vi "UHR-Fleezers Control (host) - 12.7e.vi"() -> ()   [LabVIEW 2012] (continued)
        n866 = flat-sequence {
          tunnel: w1282 -> [w1285]
          frame #0 {
            # "set paramaters (rate, volume) for flush, clear volume"
            n867 = Number To Decimal String(number="Flush rate (uL/m) P3") -> (decimal integer string=w1307:string)  [unwired: 1 in]
            n868 = local write "Inject Pump 3"(TRUE ("Inject Pump 3")) -> ()
            n869 = Concatenate Strings("irate  " ("string"), w1307, " u/m" ("string"), "\r") -> (w1309:string)
            n870 = VISA Write(VISA resource name=w1285, write buffer=w1309) -> (VISA resource name out=w1305:refnum<visa-resource-name>)  [unwired: 1 in, 2 out]
            n871 = Reciprocal(x="Flush rate (uL/m) P3") -> (1/x=w1289:dbl)
            n872 = Number To Decimal String(number="Volume (uL) P3") -> (decimal integer string=w1296:string)  [unwired: 1 in]
            n873 = Multiply(x="Volume (uL) P3", y=w1289) -> (x*y=w1288:dbl)
            n874 = Concatenate Strings("tvolume  " ("string"), w1296, " u" ("string"), "\r") -> (w1294:string)
            n875 = Multiply(x=w1288, y=60.0) -> (x*y=→"HP3 Flush Time (s)":dbl)
            n876 = VISA Write(VISA resource name=w1305, write buffer=w1294) -> (VISA resource name out=w1293:refnum<visa-resource-name>)  [unwired: 1 in, 2 out]
            n877 = Concatenate Strings("cvolume" ("string"), "\r") -> (w1292:string)
            n878 = VISA Write(VISA resource name=w1293, write buffer=w1292) -> (VISA resource name out=w1303:refnum<visa-resource-name>)  [unwired: 1 in, 2 out]
            n879 = Concatenate Strings("irun" ("string"), "\r") -> (w1301:string)
            n880 = VISA Write(VISA resource name=w1303, write buffer=w1301) -> ()  [unwired: 1 in, 3 out]
          }
          frame #1 {
            "Flushing P3" <- TRUE ("Flushing P3")
          }
        }
      }
      event "Flush Pump 1": Value Change {
        n881 = event-data() -> ()  [unwired: 7 out]
        n882 = flat-sequence {
          tunnel: [w1323] -> w1313
          tunnel: w1312 -> [w1316]
          tunnel: w1313 -> [_]
          frame #0 {
            # "set paramaters (rate, volume) for flush, clear volume"
            n883 = local write "Inject Pump 1"(TRUE ("Inject Pump 1")) -> ()
            n884 = Number To Decimal String(number="Flush rate (uL/m) P1") -> (decimal integer string=w1339:string)  [unwired: 1 in]
            n885 = Concatenate Strings("irate  " ("string"), w1339, " u/m" ("string"), "\r") -> (w1341:string)
            n886 = VISA Write(VISA resource name=w1316, write buffer=w1341) -> (VISA resource name out=w1337:refnum<visa-resource-name>)  [unwired: 1 in, 2 out]
            n887 = Reciprocal(x="Flush rate (uL/m) P1") -> (1/x=w1320:dbl)
            n888 = Number To Decimal String(number="Volume (uL) P1") -> (decimal integer string=w1328:string)  [unwired: 1 in]
            n889 = Multiply(x="Volume (uL) P1", y=w1320) -> (x*y=w1319:dbl)
            n890 = Concatenate Strings("tvolume  " ("string"), w1328, " u" ("string"), "\r") -> (w1326:string)
            n891 = Multiply(x=w1319, y=60.0) -> (x*y=→"HP1 Flush Time (s)":dbl)
            n892 = VISA Write(VISA resource name=w1337, write buffer=w1326) -> (VISA resource name out=w1325:refnum<visa-resource-name>)  [unwired: 1 in, 2 out]
            n893 = Concatenate Strings("cvolume" ("string"), "\r") -> (w1324:string)
            n894 = VISA Write(VISA resource name=w1325, write buffer=w1324) -> (VISA resource name out=w1335:refnum<visa-resource-name>)  [unwired: 1 in, 2 out]
            n895 = Concatenate Strings("irun" ("string"), "\r") -> (w1333:string)
            n896 = VISA Write(VISA resource name=w1335, write buffer=w1333) -> (VISA resource name out=w1323:refnum<visa-resource-name>)  [unwired: 1 in, 2 out]
          }
          frame #1 {
            "Flushing P1" <- TRUE ("Flushing P3")
          }
        }
      }
      event "Clear Volume": Value Change {
        n897 = event-data() -> ()  [unwired: 7 out]
        n898 = Concatenate Strings("cvolume" ("string"), "\r") -> (w1345:string)
        n899 = VISA Write(VISA resource name=w1344, write buffer=w1345) -> ()  [unwired: 1 in, 3 out]
      }
      event "Clear Volume P3": Value Change {
        n900 = event-data() -> ()  [unwired: 7 out]
        n901 = Concatenate Strings("cvolume" ("string"), "\r") -> (w1351:string)
        n902 = VISA Write(VISA resource name=w1350, write buffer=w1351) -> ()  [unwired: 1 in, 3 out]
        n903 = local write "Clear Volume P3"(FALSE ("Clear Volume P3")) -> ()
      }
      event "Clear Volume P1": Value Change {
        n904 = event-data() -> ()  [unwired: 7 out]
        n905 = Concatenate Strings("cvolume" ("string"), "\r") -> (w1356:string)
        n906 = local write "Clear Volume P1"(FALSE ("Clear Volume P1")) -> ()
        n907 = VISA Write(VISA resource name=w1355, write buffer=w1356) -> ()  [unwired: 1 in, 3 out]
      }
      event "Display On P3": Value Change {
        n908 = event-data() -> ()  [unwired: 7 out]
        n909 = Select(t="dim 100", s="Display On P3", f="dim 0") -> (s? t:f=w1362:string)
        n910 = Concatenate Strings(w1362, "\r") -> (w1364:string)
        n911 = VISA Write(VISA resource name=w1359, write buffer=w1364) -> ()  [unwired: 1 in, 3 out]
      }
      event "Display On P1": Value Change {
        n912 = event-data() -> ()  [unwired: 7 out]
        n913 = Select(t="dim 100", s="Display On P1", f="dim 0") -> (s? t:f=w1369:string)
        n914 = Concatenate Strings(w1369, "\r") -> (w1371:string)
        n915 = VISA Write(VISA resource name=w1366, write buffer=w1371) -> ()  [unwired: 1 in, 3 out]
      }
      event "Retract Pump 3": Value Change {
        n916 = event-data() -> ()  [unwired: 7 out]
        n917 = local write "Retract Pump 3"(FALSE ("Retract Pump 3")) -> ()
        n918 = case shown="True" "Retract Pump 3" {
          tunnel: w1373 -> [_ w1376]
          frame False {
          }
          frame True {
            n919 = Number To Decimal String(number="Retract Rate (uL/m)") -> (decimal integer string=w1394:string)  [unwired: 1 in]
            n920 = Concatenate Strings("wrate  " ("string"), w1394, " u/m" ("string"), "\r") -> (w1396:string)
            n921 = VISA Write(VISA resource name=w1376, write buffer=w1396) -> (VISA resource name out=w1387:refnum<visa-resource-name>)  [unwired: 1 in, 2 out]
            n922 = Number To Decimal String(number="Retract Vol 3 (uL)") -> (decimal integer string=w1389:string)  [unwired: 1 in]
            n923 = Concatenate Strings("tvolume  " ("string"), w1389, " u" ("string"), "\r") -> (w1386:string)
            n924 = VISA Write(VISA resource name=w1387, write buffer=w1386) -> (VISA resource name out=w1382:refnum<visa-resource-name>)  [unwired: 1 in, 2 out]
            n925 = Concatenate Strings("cvolume" ("string"), "\r") -> (w1383:string)
            n926 = VISA Write(VISA resource name=w1382, write buffer=w1383) -> (VISA resource name out=w1377:refnum<visa-resource-name>)  [unwired: 1 in, 2 out]
            n927 = Concatenate Strings("wrun" ("string"), "\r") -> (w1378:string)
            n928 = VISA Write(VISA resource name=w1377, write buffer=w1378) -> ()  [unwired: 1 in, 3 out]
          }
        }
      }
      event "Retract Pump 1": Value Change {
        n929 = event-data() -> ()  [unwired: 7 out]
        n930 = local write "Retract Pump 1"(FALSE ("Retract Pump 1")) -> ()
        n931 = case shown="True" "Retract Pump 1" {
          tunnel: w1398 -> [_ w1403]
          frame False {
          }
          frame True {
            n932 = local read "Retract Rate (uL/m)"() -> (w1401:dbl)
            n933 = Number To Decimal String(number=w1401) -> (decimal integer string=w1419:string)  [unwired: 1 in]
            n934 = Concatenate Strings("wrate  " ("string"), w1419, " u/m" ("string"), "\r") -> (w1421:string)
            n935 = VISA Write(VISA resource name=w1403, write buffer=w1421) -> (VISA resource name out=w1413:refnum<visa-resource-name>)  [unwired: 1 in, 2 out]
            n936 = Number To Decimal String(number="Retract Vol 1 (uL)") -> (decimal integer string=w1415:string)  [unwired: 1 in]
            n937 = Concatenate Strings("tvolume  " ("string"), w1415, " u" ("string"), "\r") -> (w1412:string)
            n938 = VISA Write(VISA resource name=w1413, write buffer=w1412) -> (VISA resource name out=w1409:refnum<visa-resource-name>)  [unwired: 1 in, 2 out]
            n939 = Concatenate Strings("cvolume" ("string"), "\r") -> (w1410:string)
            n940 = VISA Write(VISA resource name=w1409, write buffer=w1410) -> (VISA resource name out=w1404:refnum<visa-resource-name>)  [unwired: 1 in, 2 out]
            n941 = Concatenate Strings("wrun" ("string"), "\r") -> (w1405:string)
            n942 = VISA Write(VISA resource name=w1404, write buffer=w1405) -> ()  [unwired: 1 in, 3 out]
          }
        }
      }
      event "Flip Green Filter": Value Change {
        n943 = event-data() -> ()  [unwired: 7 out]
        n944 = Not(x="Flip Green Filter") -> (.not. x?=w1424:bool)
        n945 = local write "Flip Green Filter"(w1424) -> ()
        n946 = flat-sequence {
          tunnel: [w1433] -> w1429
          tunnel: [w1432] -> w1428
          tunnel: w1423 -> [w1431]
          tunnel: [w1436] -> w1427
          tunnel: w1429 -> [w1436]
          tunnel: [w1435] -> w1426
          tunnel: w1428 -> [w1435]
          tunnel: w1427 -> [w1440]
          tunnel: w1426 -> [w1439]
          tunnel: [w1438] -> w1430
          frame #0 {
            n947 = xnode "Read/Write Control"("FPGA VI Reference In"=w1431, "Green Filter Flipper"=TRUE) -> ("FPGA VI Reference Out"=w1433:T20, "error out"=w1432:errorcluster)  [unwired: 1 in]
          }
          frame #1 {
            n948 = Wait (ms)(milliseconds to wait=u32 100) -> ()  [unwired: 1 out]
          }
          frame #2 {
            n949 = xnode "Read/Write Control"("FPGA VI Reference In"=w1440, "error in"=w1439, "Green Filter Flipper"=FALSE) -> ("error out"=w1438:errorcluster)  [unwired: 1 out]
          }
        }
      }
      event "Pump 1 contents", "Pump 3 contents": Value Change {
        n950 = event-data() -> ()  [unwired: 7 out]
        n951 = local read "Pump 1 contents"() -> (→"Pump 1 cont disp":string)
        n952 = local read "Pump 3 contents"() -> (→"Pump 3 cont disp":string)
      }
      event "Reset Trap Pos. FB": Value Change {
        n953 = event-data() -> ()  [unwired: 7 out]
        n954 = xnode "Read/Write Control"("FPGA VI Reference In"=w1444, "Trap Pos. FB Reset"="Reset Trap Pos. FB") -> ()  [unwired: 1 in, 2 out]
      }
      event "Rem fb disp offset": Value Change {
        n955 = event-data() -> ()  [unwired: 7 out]
        n956 = local write "Rem fb disp offset"(FALSE ("Rem fb disp offset")) -> ()
        n957 = local read "Mean T1 Position (nm)"() -> (w1447:dbl)
        n958 = local read "FB Trap Pos Offset"() -> (w1448:dbl)
        n959 = Subtract(x=w1448, y=w1447) -> (x-y=w1446:dbl)
        n960 = local write "FB Trap Pos Offset"(w1446) -> ()
      }
      event "Threshold (nm)": Value Change {
        n961 = event-data() -> ()  [unwired: 7 out]
        n962 = flat-sequence {
          tunnel: [w1453] -> w1451
          tunnel: w1450 -> [w1452]
          tunnel: w1451 -> [w1464]
          frame #0 {
            n963 = xnode "Read/Write Control"("FPGA VI Reference In"=w1452) -> ("FPGA VI Reference Out"=w1456:T20, "error out"=w1455:errorcluster, "FPGA TTrig Thresh"=w1457:i64)  [unwired: 1 in]
            n964 = local read "Threshold stored (nm)"() -> (w1463:dbl)
            n965 = local read "Threshold (nm)"() -> (w1453:dbl)
            n966 = local read "AOM X Cal (nm/MHz)"() -> (w1461:dbl)
            n967 = Subtract(x=w1453, y=w1463) -> (x-y=w1462:dbl)
            n968 = Divide(x=w1462, y=w1461) -> (x/y=w1459:dbl)
            n969 = call "IR AOM freq to word.vi"("Frequency In (MHz)"=w1459) -> ("Frequency Word Out (double)"=w1460:dbl)
            n970 = To Quad Integer(1:w1460) -> (0:w1458:i64)
            n971 = Add(x=w1457, y=w1458) -> (x+y=w1454:i64)
            n972 = xnode "Read/Write Control"("FPGA VI Reference In"=w1456, "error in"=w1455, "FPGA TTrig Thresh"=w1454) -> ()  [unwired: 2 out]
          }
          frame #1 {
            "Threshold stored (nm)" <- w1464
          }
        }
      }
      event "FB Trig Integrate": Value Change {
        n973 = event-data() -> ()  [unwired: 7 out]
        n974 = local read "FB Trig Integrate"() -> (w1467:u32)
        n975 = xnode "Read/Write Control"("FPGA VI Reference In"=w1465, "FB Trig Integrate"=w1467) -> ("error out"=w1466:errorcluster)  [unwired: 1 in, 1 out]
      }
      event "11": Value Change {
        n976 = event-data() -> ()  [unwired: 7 out]
        n977 = local read "11"() -> (w1468:bool)
        n978 = case shown="True" w1468 {
          frame False {
          }
          frame True {
            n979 = local read "Messages"() -> (w1470:string)
            n980 = call "Update messages.vi"("Message to add"="You kicked it up to 11!", "Old message string"=w1470) -> ("New message string"=w1471:string)
            n981 = call <vilib>:"Beep.vi"() -> ()  [unwired: 12 in]
            n982 = local write "Messages"(w1471) -> ()
          }
        }
      }
      event "Trap Pos. FB ON": Value Change {
        n983 = event-data() -> ()  [unwired: 7 out]
        n984 = xnode "Read/Write Control"("FPGA VI Reference In"=w1472, "Force feedback"="Trap Pos. FB ON") -> ()  [unwired: 1 in, 2 out]
      }
      event "Remove Action Offset": Value Change {
        n985 = event-data() -> ()  [unwired: 7 out]
        n986 = local write "Remove Action Offset"(FALSE ("Remove Action Offset")) -> ()
        n987 = local read "Trap Pos. FB Mult Factor"() -> (w1479:i64)
        n988 = local read "Trap Pos FB Action"() -> (w1477:i64)
        n989 = local read "Trap Pos. FB Offset Factor"() -> (w1475:i64)
        n990 = Multiply(x=w1479, y=w1477) -> (x*y=w1478:i64)
        n991 = Add(x=w1478, y=w1475) -> (x+y=w1476:i64)
        n992 = local write "Trap Pos. FB Offset Factor"(w1476) -> ()
        n993 = xnode "Read/Write Control"("FPGA VI Reference In"=w1474, "Trap Pos. FB Offset Factor"=w1476) -> ()  [unwired: 1 in, 2 out]
      }
      event "Remove Unwinding Offset": Value Change {
        n994 = event-data() -> ()  [unwired: 7 out]
        n995 = local write "Remove Unwinding Offset"(FALSE ("Remove Action Offset")) -> ()
        n996 = local read "Trap Pos. FB Mult Factor"() -> (w1493:i64)
        n997 = local read "Trap Pos FB Action"() -> (w1491:i64)
        n998 = local read "Trap Pos. FB Offset Factor"() -> (w1490:i64)
        n999 = Multiply(x=w1493, y=w1491) -> (x*y=w1492:i64)
        n1000 = local read "Trap Pos. FB Mult Factor"() -> (w1489:i64)
        n1001 = Add(x=w1492, y=w1490) -> (x+y=w1483:i64)
        n1002 = Multiply(x=32768, y="factor") -> (x*y=w1486:dbl)
        n1003 = Multiply(x=w1486, y=w1489) -> (x*y=w1488:dbl)
        n1004 = Subtract(x=w1483, y=w1488) -> (x-y=w1487:dbl)
        n1005 = To Quad Integer(1:w1487) -> (0:w1482:i64)
        n1006 = xnode "Read/Write Control"("FPGA VI Reference In"=w1481, "Trap Pos. FB Offset Factor"=w1482) -> ()  [unwired: 1 in, 2 out]
        n1007 = local write "Trap Pos. FB Offset Factor"(w1482) -> ()
      }
      event "Trap Pos. FB Range", "Trap Pos. FB Gains", "Trap Pos. FB Mult Factor", "Trap Pos. FB Offset Factor", "Trap Pos FB Negate Action", "Trap Pos FB Monitor\nT1 or T2", "Differential FB?", "Negate Diff?": Value Change {
        n1008 = event-data() -> ()  [unwired: 7 out]
        n1009 = Unbundle By Name("Trap Pos. FB Gains") -> ("proportional gain (Kc)"=w1498:fxp<+/-,16,8>, "integral gain (Kc*Ts/Ti)"=w1497:fxp<+/-,16,8>, "derivative gain (Kc*Td/Ts)"=w1496:fxp<+/-,16,8>)
        n1010 = local read "Negate Diff?"() -> (w1503:bool)
        n1011 = Unbundle By Name("Trap Pos. FB Range") -> ("output high"=w1501:fxp<+/-,16,1>, "output low"=w1500:fxp<+/-,16,1>)
        n1012 = xnode "Read/Write Control"("FPGA VI Reference In"=w1495, "FB2 output high"=w1501, "FB2 output low"=w1500, "P2"=w1498, "I2"=w1497, "D2"=w1496, "Trap Pos. FB Mult Factor"="Trap Pos. FB Mult Factor", "Trap Pos. FB Offset Factor"="Trap Pos. FB Offset Factor", "Trap Pos FB Negate Action"="Trap Pos FB Negate Action", "Trap Pos FB Monitor T1 or T2"="Trap Pos FB Monitor\nT1 or T2", "AI1 X Scale"="Trap Pos. AI1 X Pre-scale", "Negate Diff?"=w1503, "Diff FB Measurement?"="Differential FB?") -> ()  [unwired: 1 in, 2 out]
      }
      event "Trap Pos FB SP", "Trap Pos FB SP 2", "Use SP 2": Value Change {
        n1013 = event-data() -> ()  [unwired: 7 out]
        n1014 = Select(t="Trap Pos FB SP 2", s="Use SP 2", f="Trap Pos FB SP") -> (s? t:f=w1511:fxp<+/-,16,1>)
        n1015 = xnode "Read/Write Control"("FPGA VI Reference In"=w1510, "Trap Pos. FB SP"=w1511) -> ()  [unwired: 1 in, 2 out]
      }
      event "Offset SP2 from SP1": Value Change {
        n1016 = event-data() -> ()  [unwired: 7 out]
        n1017 = local read "Trap Pos FB SP"() -> (w1517:fxp<+/-,16,1>)
        n1018 = Add(x=w1517, y="SP2 Offset") -> (x+y=w1515:fxp<+/-,16,1>)
        n1019 = property on="Trap Pos FB SP 2" class="DigNum (strict)"("Val(Sgnl)"=w1515) -> ()  [unwired: 2 in, 2 out]
        n1020 = local write "Offset SP2 from SP1"(FALSE ("Offset SP2 from SP1")) -> ()
      }
      event "Set Reading to\nSetpoint": Value Change {
        # "This is the actual PID input signal"
        n1021 = event-data() -> ()  [unwired: 7 out]
        n1022 = local write "Set Reading to\nSetpoint"(FALSE ("Set SP to Reading")) -> ()
        n1023 = xnode "Read/Write Control"("FPGA VI Reference In"=w1519) -> ("FPGA VI Reference Out"=w1522:T20, "error out"=w1521:errorcluster, "Trap Pos FB Int-Norm Signal"=w1520:fxp<+/-,16,1>)  [unwired: 1 in]
        n1024 = local read "Differential FB?"() -> (w1523:bool)
        n1025 = case shown="False" w1523 {
          tunnel: [w1528 w1535] -> w1525
          tunnel: w1520 -> [w1526 w1535]
          frame False {
            n1026 = local read "Trap Pos FB Monitor\nT1 or T2"() -> (w1531:bool)
            n1027 = local read "Trap X AI1 (DMA)"() -> (w1534:T13)
            n1028 = Unbundle By Name(w1534) -> ("Set 1"=w1533:fxp<+/-,16,1>, "Set 2"=w1532:fxp<+/-,16,1>)
            n1029 = Select(t=w1533, s=w1531, f=w1532) -> (s? t:f=w1530:fxp<+/-,16,1>)
            n1030 = Not(x="Set SP Using...") -> (.not. x?=w1527:bool)
            n1031 = Select(t=w1526, s=w1527, f=w1530) -> (s? t:f=w1528:fxp<+/-,16,1>)
          }
          frame True {
          }
        }
        n1032 = xnode "Read/Write Control"("FPGA VI Reference In"=w1522, "error in"=w1521, "Trap Pos. FB SP"=w1525) -> ()  [unwired: 2 out]
        n1033 = local write "Trap Pos FB SP"(w1525) -> ()
      }
      event "Trap Pos. FB Out Scale 2^n": Value Change {
        n1034 = event-data() -> ()  [unwired: 7 out]
        n1035 = Scale By Power Of 2(n="Trap Pos. FB Out Scale 2^n", x=ext 1.0) -> (x*2^n=w1536:ext)
        n1036 = property on="Trap Pos. FB Mult Factor" class="DigNum (strict)"("Val(Sgnl)"=w1536) -> ()  [unwired: 2 in, 2 out]
      }
      event "Trap Pos FB Int Count": Value Change {
        n1037 = event-data() -> ()  [unwired: 7 out]
        n1038 = xnode "Read/Write Control"("FPGA VI Reference In"=w1539, "Trap Pos FB Int Count"="Trap Pos FB Int Count") -> ()  [unwired: 1 in, 2 out]
      }
      event "Trap pos": Value Change {
        n1039 = event-data() -> ()  [unwired: 7 out]
        n1040 = case shown="True" "Trap pos" {
          frame False {
            n1041 = property on="Trap Delta Graph" class="WFGraph (strict)"("Visible"=TRUE) -> ()  [unwired: 2 in, 2 out]
            n1042 = property on="Saved trap pos" class="WFGraph (strict)"("Visible"=FALSE) -> ()  [unwired: 2 in, 2 out]
          }
          frame True {
            n1043 = property on="Saved trap pos" class="WFGraph (strict)"("Visible"=TRUE) -> ()  [unwired: 2 in, 2 out]
            n1044 = property on="Trap Delta Graph" class="WFGraph (strict)"("Visible"=FALSE) -> ()  [unwired: 2 in, 2 out]
          }
        }
      }
    }
    "error out 2" <- w406
    n1045 = node-c288() -> ()  [unwired: 2 out]
  }
  n1046 = timed-loop "Rough control of MCL mirror stage (debugging)" {
    tunnel: [w1548] -> w76
    timing: w22 -> [_]
    timing-out: [_] -> w21
    tunnel: w5 -> [w1546]
    stop <- w1548 stop-if-true
    n1047 = node-c288() -> ()  [unwired: 2 out]
    n1048 = case shown="2" "MCL Mode" {
      tunnel: w1546 -> [_ w1551 w1598]
      frame 0, Default {
      }
      frame 1 {
        n1049 = node-c288() -> (w1553:T23)  [unwired: 4 out]
        n1050 = timed-loop "Oscillate MCL mirror" {
          timing: w1553 -> [_]
          timing-out: [_] -> w1552
          tunnel: w1551 -> [w1554]
          i -> [w1592]
          stop <- w1555 stop-if-true
          n1051 = node-c288() -> (w1591:i64)  [unwired: 1 out]
          n1052 = Multiply(x="AO1", y=32767.0) -> (x*y=w1587:dbl)
          n1053 = Multiply(x="AO2", y=32767.0) -> (x*y=w1582:dbl)
          n1054 = Divide(x=w1587, y=10.0) -> (x/y=w1588:dbl)
          n1055 = Divide(x=w1582, y=10.0) -> (x/y=w1583:dbl)
          n1056 = To Word Integer(number=w1588) -> (16bit integer=w1580:i16)
          n1057 = To Word Integer(number=w1583) -> (16bit integer=w1579:i16)
          n1058 = Divide(x=w1591, y=i64 1000) -> (x/y=w1562:dbl)
          n1059 = Multiply(x=w1562, y=w1592) -> (x*y=w1573:dbl)
          n1060 = Multiply(x="Osc. freq. (Hz) 2", y=6.283185307179586) -> (x*y=w1574:dbl)
          n1061 = Multiply(x=w1574, y=w1573) -> (x*y=w1572:dbl)
          n1062 = Sine(x=w1572) -> (sin(x)=w1571:dbl)
          n1063 = Multiply(x=w1571, y="Osc. amp. (V)") -> (x*y=w1569:dbl)
          n1064 = Add(x=w1569, y="Osc. center (V)") -> (x+y=w1567:dbl)
          n1065 = Divide(x=w1567, y=10.0) -> (x/y=w1565:dbl)
          n1066 = Multiply(x=w1565, y=32767.0) -> (x*y=w1560:dbl)
          n1067 = Select(t=w1560, s="Scan axis", f=w1580) -> (s? t:f=w1578:dbl)
          n1068 = Select(t=w1579, s="Scan axis", f=w1560) -> (s? t:f=w1577:dbl)
          n1069 = local read "MCL Mode"() -> (w1559:u16)
          n1070 = Not Equal?(x=w1559, y=u16 1) -> (x != y?=w1556:bool)
          n1071 = local read "Stop All"() -> (w1557:bool)
          n1072 = xnode "Read/Write Control"("FPGA VI Reference In"=w1554, "AO1"=w1578, "AO2"=w1577) -> ()  [unwired: 1 in, 2 out]
          n1073 = Compound Arithmetic op=OR(w1557, w1556) -> (w1555:bool)
          n1074 = node-c288() -> ()  [unwired: 2 out]
        }
        n1075 = node-c288(w1552) -> ()  [unwired: 1 out]
      }
      frame 2 {
        n1076 = case shown="True" "Start Scan" {
          tunnel: w1598 -> [_ w1600]
          frame False {
          }
          frame True {
            n1077 = Subtract(x="End (V)", y="Begin (V)") -> (x-y=w1607:dbl)
            n1078 = Decrement(x="N Points") -> (x-1=w1606:dbl)
            n1079 = Divide(x=w1607, y=w1606) -> (x/y=w1604:dbl)
            n1080 = for {
              N: "N Points" -> [_]
              tunnel: "Begin (V)" -> [w1623]
              tunnel: [w1615] -> w1610 mode=indexing
              tunnel: w1604 -> [w1614]
              tunnel: [w1612] -> w1603 mode=indexing
              tunnel: w1600 -> [w1611]
              i -> [w1622]
              n1081 = Multiply(x=w1614, y=w1622) -> (x*y=w1621:dbl)
              n1082 = Add(x=w1623, y=w1621) -> (x+y=w1618:dbl)
              n1083 = local read "Scan axis"() -> (w1613:bool)
              n1084 = local read "AO1"() -> (w1620:dbl)
              n1085 = local read "AO2"() -> (w1619:dbl)
              n1086 = Select(t=w1618, s=w1613, f=w1620) -> (s? t:f=w1617:dbl)
              n1087 = Select(t=w1619, s=w1613, f=w1618) -> (s? t:f=w1616:dbl)
              n1088 = flat-sequence {
                tunnel: w1617 -> [w1627]
                tunnel: w1616 -> [w1626]
                tunnel: w1611 -> [w1624]
                tunnel: [w1637] -> w1615
                tunnel: [w1636] -> w1612
                frame #0 {
                  w1630 = 10.0 ("y")
                  w1625 = 32767.0 ("y")
                  n1089 = Multiply(x=w1627, y=w1625) -> (x*y=w1633:dbl)
                  n1090 = Multiply(x=w1626, y=w1625) -> (x*y=w1631:dbl)
                  n1091 = Divide(x=w1633, y=w1630) -> (x/y=w1634:dbl)
                  n1092 = Divide(x=w1631, y=w1630) -> (x/y=w1632:dbl)
                  n1093 = To Word Integer(number=w1634) -> (16bit integer=w1628:i16)
                  n1094 = To Word Integer(number=w1632) -> (16bit integer=w1629:i16)
                  n1095 = xnode "Read/Write Control"("FPGA VI Reference In"=w1624, "AO1"=w1628, "AO2"=w1629) -> ()  [unwired: 1 in, 2 out]
                }
                frame #1 {
                  n1096 = Wait (ms)(milliseconds to wait="DAQ Delay (ms)") -> ()  [unwired: 1 out]
                }
                frame #2 {
                  n1097 = local read "Slow mean"() -> (w1637:dbl)
                  n1098 = local read "Sigma"() -> (w1636:dbl)
                }
              }
            }
            n1099 = Bundle("Begin (V)"="Begin (V)", w1604, w1610) -> (→"MCL Scan":cluster{"Begin (V)":dbl, dbl, dbl[]})  [unwired: 1 out]
            n1100 = Bundle("Begin (V)"="Begin (V)", w1604, w1603) -> (→"MCL Scan 2":cluster{"Begin (V)":dbl, dbl, dbl[]})  [unwired: 1 out]
          }
        }
      }
    }
    n1101 = local read "Stop All"() -> (w1548:bool)
    n1102 = node-c288() -> ()  [unwired: 2 out]
  }
  n1103 = timed-loop "Run Scripts, including: stage motion" {
    tunnel: w59 -> [w1646]
    tunnel: w58 -> [w1647]
    tunnel: [w1647] -> w57
    tunnel: [w1646] -> w56
    timing: w54 -> [_]
    timing-out: [_] -> w53
    tunnel: w42 -> [w1645]
    tunnel: w43 -> [w1644]
    tunnel: w32 -> [w1641]
    tunnel: w31 -> [w1640]
    tunnel: w30 -> [w1642]
    tunnel: w29 -> [w1643]
    tunnel: w17 -> [w1639]
    tunnel: w5 -> [w1638]
    stop <- w1648 stop-if-true
    n1104 = node-c288() -> ()  [unwired: 1 in, 1 out]
    n1105 = event shown="[22] \"Move in a Circle\": Value Change" {
      selector: _ -> [_ _ _ _ _ _ _ _ _ _ _ _ _ _ _ _ _ _ _ _ _ _ _ _]
      dyn-events: _ -> [_ _ _ _ _ _ _ _ _ _ _ _ _ _ _ _ _ _ _ _ _ _ _ _]
      timeout: _ -> [_ _ _ _ _ _ _ _ _ _ _ _ _ _ _ _ _ _ _ _ _ _ _ _]
      tunnel: ["Set Position" "Move to Position" _ _ _ _ _ _ "Read Harvard" _ _ _ _ _ _ "Got ADig bead" "Force FB Data\nScript" _ "Got DNA bead" "Take Stepping Data" _ "Take Detection Laser\nImage" _ _] -> _
      tunnel: [_ _ _ _ _ _ _ _ _ _ _ _ _ _ _ _ _ _ _ _ _ _ _ w2472] -> w1648
      tunnel: w1646 -> [w1666 w1674 w1687 w1717 _ _ _ _ _ w1833 w1873 w1954 w1983 w2115 w2141 _ w2177 _ _ _ _ _ _ _]
      tunnel: w1647 -> [w1667 w1675 w1688 w1718 _ _ _ _ _ w1834 w1874 w1955 w1984 w2116 w2142 _ w2178 _ _ _ _ _ _ _]
      tunnel: w1645 -> [_ _ _ _ _ _ _ _ w1818 _ _ _ _ _ _ _ _ _ _ _ _ _ _ _]
      tunnel: w1644 -> [_ _ _ _ _ _ _ _ w1817 _ _ _ _ _ _ _ _ _ _ _ _ _ _ _]
      tunnel: w1643 -> [_ _ _ _ _ _ _ _ _ _ _ _ _ _ _ _ _ _ _ _ _ _ _ _]
      tunnel: w1642 -> [_ _ _ _ _ _ _ _ _ _ _ _ _ _ _ _ _ _ _ _ _ _ _ _]
      tunnel: w1641 -> [_ _ _ _ _ _ _ _ _ _ _ _ _ _ _ _ _ _ _ _ _ _ _ _]
      tunnel: w1640 -> [_ _ _ _ _ _ _ _ _ _ _ _ _ _ _ _ _ _ _ _ _ _ _ _]
      tunnel: w1639 -> [_ _ _ _ w1745 w1773 w1797 w1808 _ _ _ _ _ _ _ _ _ _ _ _ _ _ _ w2471]
      tunnel: w1638 -> [_ _ _ _ _ _ _ _ _ _ _ _ _ _ _ _ _ _ _ _ _ _ w2338 _]
      event "Set Position", "Set Position 2", "Set Position 3", "Set Position 4", "Set Position 5", "Set Position 1": Value Change {
        n1106 = event-data() -> ()  [unwired: 1 in, 5 out]
        n1107 = Build Array("Set Position 1", "Set Position 2", "Set Position 3", "Set Position 4", "Set Position 5") -> (w1665:bool[])
        n1108 = Boolean Array To Number(Boolean array=w1665) -> (number=w1664:u32)
        n1109 = Logarithm Base 2(1:w1664) -> (0:w1656:dbl)
        n1110 = call "Read Stage Position.vi"("error in"=w1666, "VISA resource name in"=w1667) -> ("Current Position"=w1671:cluster{dbl, dbl, dbl}, "error out"=w1670:errorcluster)  [unwired: 2 out]
        n1111 = Decrement(x="Position") -> (x-1=w1654:dbl)
        n1112 = Greater Or Equal?(x=w1656, y=0.0) -> (x >= y?=w1657:bool)
        n1113 = Cluster To Array(cluster=w1671) -> (array=w1668:dbl[])
        n1114 = local write "Stage Control Serial Error"(w1670) -> ()
        n1115 = Select(t=w1656, s=w1657, f=w1654) -> (s? t:f=w1653:dbl)
        n1116 = Increment(x=w1653) -> (x+1=w1652:dbl)
        n1117 = Build Array (concatenate)(w1652, w1668) -> (w1651:dbl[])
        n1118 = Replace Array Subset(array="Saved Stage Positions", new element=w1651, index (row)=w1653) -> (w1669:dbl[][])  [unwired: 1 in]
        n1119 = local write "Saved Stage Positions"(w1669) -> ()
      }
      event "Move to Position": Value Change {
        n1120 = event-data() -> ()  [unwired: 1 in, 5 out]
        n1121 = flat-sequence {
          tunnel: w1675 -> [w1679]
          tunnel: w1674 -> [w1678]
          frame #0 {
            n1122 = local read "Saved Stage Positions"() -> (w1681:dbl[][])
            n1123 = local read "Position"() -> (w1680:dbl)
            n1124 = local write "Stage Moving"(TRUE ("Stage Moving")) -> ()
            n1125 = call "move to saved stage position.vi"("error in"=w1678, "Stage VISA resource name in"=w1679, "Position"=w1680, "Saved Stage Positions"=w1681) -> ("error out"=w1677:errorcluster)  [unwired: 1 out]
            n1126 = local write "Stage Control Serial Error"(w1677) -> ()
          }
          frame #1 {
            n1127 = call <vilib>:"Beep.vi"() -> ()  [unwired: 3 in, 9 out]
            n1128 = local write "Stage Moving"(FALSE ("Stage Moving")) -> ()
          }
        }
      }
      event "Move Cap. 1 (DNA Bottom)": Value Change {
        n1129 = event-data() -> ()  [unwired: 1 in, 5 out]
        n1130 = local write "Move Cap. 1 (DNA Bottom)"(FALSE ("Move Cap. 1 (DNA Right)")) -> ()
        n1131 = flat-sequence {
          tunnel: w1687 -> [w1690]
          tunnel: w1688 -> [w1691]
          tunnel: [w1691] -> w1685
          tunnel: [w1690] -> w1684
          tunnel: w1685 -> [w1693]
          tunnel: w1684 -> [w1692]
          frame #0 {
            n1132 = property on="Sample Channel\nFlow" class="Bool (strict)"("Val(Sgnl)"="Cap 1 Samp Flow ON") -> ()  [unwired: 2 in, 2 out]
          }
          frame #1 {
            n1133 = local read "Saved Stage Positions"() -> (w1703:dbl[][])
            n1134 = local write "Stage Moving"(TRUE ("Stage Moving")) -> ()
            n1135 = Array Subset(array=w1703, index (row)=0 ("index"), length (row)=1 ("length"), index (col)=1 ("index"), length (col)=3 ("length")) -> (w1700:dbl[][])
            n1136 = Reshape Array(w1700, 3 ("dimension size")) -> (w1698:dbl[])
            n1137 = Array To Cluster(array=w1698) -> (cluster=w1697:cluster{"[0]":dbl, "[1]":dbl, "[2]":dbl})
            n1138 = call "Set Stage Position.vi"("Position"=w1697, "error in"=w1692, "VISA resource name in"=w1693) -> ("error out"=w1696:errorcluster)  [unwired: 2 out]
            n1139 = local write "Stage Control Serial Error"(w1696) -> ()
          }
          frame #2 {
            n1140 = local write "Stage Moving"(FALSE ("Stage Moving")) -> ()
            n1141 = case shown="True" "Cap 1 Flow ON" {
              frame False {
              }
              frame True {
                n1142 = property on="Inject Pump 1" class="Bool (strict)"("Val(Sgnl)"=TRUE ("Value (Signaling)")) -> ()  [unwired: 2 in, 2 out]
              }
            }
            n1143 = call <vilib>:"Beep.vi"() -> ()  [unwired: 3 in, 9 out]
          }
          frame #3 {
            n1144 = property on="Sample Channel\nFlow" class="Bool (strict)"("Val(Sgnl)"=FALSE ("Value (Signaling)")) -> ()  [unwired: 2 in, 2 out]
            n1145 = local read "Cap. 2 BD T1?\n(ADig T1, DNA T2)"() -> (w1710:bool)
            n1146 = case shown="True" w1710 {
              tunnel: "Cap 1 T ON" -> [w1712 w1713]
              frame False {
                n1147 = property on="Trap 1 (ON/OFF)" class="Bool (strict)"("Val(Sgnl)"=w1712) -> ()  [unwired: 2 in, 2 out]
              }
              frame True {
                n1148 = property on="Trap 2 (ON/OFF)" class="Bool (strict)"("Val(Sgnl)"=w1713) -> ()  [unwired: 2 in, 2 out]
              }
            }
            n1149 = property on="Got DNA bead" class="Bool"("Key Focus"=TRUE) -> ()  [unwired: 2 in, 2 out]
          }
        }
      }
      event "Move Cap. 2 (ADig Top)": Value Change {
        n1150 = event-data() -> ()  [unwired: 1 in, 5 out]
        n1151 = local write "Move Cap. 2 (ADig Top)"(FALSE ("Move Cap. 2 (ADig Left)")) -> ()
        n1152 = flat-sequence {
          tunnel: w1717 -> [w1720]
          tunnel: w1718 -> [w1721]
          tunnel: [w1721] -> w1715
          tunnel: [w1720] -> w1714
          tunnel: w1715 -> [w1724]
          tunnel: w1714 -> [w1723]
          frame #0 {
            n1153 = property on="Sample Channel\nFlow" class="Bool (strict)"("Val(Sgnl)"="Cap 2 Samp Flow ON") -> ()  [unwired: 2 in, 2 out]
          }
          frame #1 {
            w1722 = FALSE ("Value (Signaling)")
            n1154 = local read "Saved Stage Positions"() -> (w1734:dbl[][])
            n1155 = local write "Stage Moving"(TRUE ("Stage Moving")) -> ()
            n1156 = Array Subset(array=w1734, index (row)=1 ("index"), length (row)=1 ("length"), index (col)=1 ("index"), length (col)=3 ("length")) -> (w1731:dbl[][])
            n1157 = Reshape Array(w1731, 3 ("dimension size")) -> (w1729:dbl[])
            n1158 = property on="Trap 1 (ON/OFF)" class="Bool (strict)"("Val(Sgnl)"=w1722) -> ()  [unwired: 2 in, 2 out]
            n1159 = property on="Trap 1 (ON/OFF)" class="Bool (strict)"("Val(Sgnl)"=w1722) -> ()  [unwired: 2 in, 2 out]
            n1160 = Array To Cluster(array=w1729) -> (cluster=w1728:cluster{"[0]":dbl, "[1]":dbl, "[2]":dbl})
            n1161 = call "Set Stage Position.vi"("Position"=w1728, "error in"=w1723, "VISA resource name in"=w1724) -> ("error out"=w1727:errorcluster)  [unwired: 2 out]
            n1162 = local write "Stage Control Serial Error"(w1727) -> ()
          }
          frame #2 {
            n1163 = local write "Stage Moving"(FALSE ("Stage Moving")) -> ()
            n1164 = call <vilib>:"Beep.vi"() -> ()  [unwired: 3 in, 9 out]
            n1165 = case shown="True" "Cap 2 Flow ON" {
              frame False {
              }
              frame True {
                n1166 = property on="Inject Pump 3" class="Bool (strict)"("Val(Sgnl)"=TRUE ("Value (Signaling)")) -> ()  [unwired: 2 in, 2 out]
              }
            }
          }
          frame #3 {
            n1167 = property on="Sample Channel\nFlow" class="Bool (strict)"("Val(Sgnl)"=FALSE ("Value (Signaling)")) -> ()  [unwired: 2 in, 2 out]
            n1168 = case shown="False" "Cap. 2 BD T1?\n(ADig T1, DNA T2)" {
              tunnel: "Cap 2 T ON" -> [w1743 w1744]
              frame False {
                n1169 = property on="Trap 2 (ON/OFF)" class="Bool (strict)"("Val(Sgnl)"=w1743) -> ()  [unwired: 2 in, 2 out]
              }
              frame True {
                n1170 = property on="Trap 1 (ON/OFF)" class="Bool (strict)"("Val(Sgnl)"=w1744) -> ()  [unwired: 2 in, 2 out]
              }
            }
            n1171 = property on="Got ADig bead" class="Bool"("Key Focus"=TRUE) -> ()  [unwired: 2 in, 2 out]
          }
        }
      }
      event "Initialize Blue Laser": Value Change {
        n1172 = event-data() -> ()  [unwired: 1 in, 5 out]
        n1173 = flat-sequence {
          tunnel: w1745 -> [w1764]
          frame #0 {
            n1174 = Concatenate Strings("slmp ", "Blue Laser\nModulation\nPower (mW)") -> (w1763:string)
            n1175 = call "serial write macro.vi"("String"=w1763, "Delay (ms)"="Delay (ms)", "VISA resource name"=w1764) -> ("read buffer"=w1752:string, "error out"=w1753:errorcluster, "VISA resource name out"=w1760:refnum<visa-resource-name>)
            n1176 = local write "read blue buffer"(w1752) -> ()
            n1177 = local write "Blue Error Out"(w1753) -> ()
            n1178 = call "serial write macro.vi"("String"="sdmes 1", "Delay (ms)"="Delay (ms)", "VISA resource name"=w1760) -> ("read buffer"=w1750:string, "error out"=w1751:errorcluster, "VISA resource name out"=w1758:refnum<visa-resource-name>)
            n1179 = local write "Blue Error Out"(w1751) -> ()
            n1180 = local write "read blue buffer"(w1750) -> ()
            n1181 = call "serial write macro.vi"("String"="sames 1", "Delay (ms)"="Delay (ms)", "VISA resource name"=w1758) -> ("read buffer"=w1747:string, "error out"=w1749:errorcluster, "VISA resource name out"=w1755:refnum<visa-resource-name>)
            n1182 = local write "read blue buffer"(w1747) -> ()
            n1183 = local write "Blue Error Out"(w1749) -> ()
            n1184 = call "serial write macro.vi"("String"="l1", "Delay (ms)"="Delay (ms)", "VISA resource name"=w1755) -> ("read buffer"=w1746:string, "error out"=w1748:errorcluster)  [unwired: 1 out]
            n1185 = local write "read blue buffer"(w1746) -> ()
            n1186 = local write "Blue Error Out"(w1748) -> ()
          }
          frame #1 {
            n1187 = local write "Initialize Blue Laser"(FALSE ("Initialize")) -> ()
          }
        }
      }
      event "Blue Laser Modluation Mode": Value Change {
        # "Changes the type of modulation for the blue laser"
        n1188 = event-data() -> ()  [unwired: 1 in, 5 out]
        n1189 = case shown="\"Constant Power\"" "Blue Laser Modluation Mode" {
          tunnel: ["sdmes 1" w1782 "sdmes 1" "sdmes 0"] -> w1767
          tunnel: ["sames 1" "cp" "sames 0" "sames 1"] -> w1766
          frame "Digital + Analog", Default {
          }
          frame "Constant Power" {
            n1190 = local read "Blue Laser\nModulation\nPower (mW)"() -> (w1785:string)
            n1191 = Decimal String To Number(string=w1785) -> (number=w1781:i32)  [unwired: 2 in, 1 out]
            n1192 = Divide(x=w1781, y=1000) -> (x/y=w1779:dbl)
            n1193 = Number To Fractional String(number=w1779) -> (F-format string=w1780:string)  [unwired: 3 in]
            n1194 = Concatenate Strings("p ", w1780) -> (w1782:string)
          }
          frame "Digital Only" {
          }
          frame "Analog Only" {
          }
        }
        n1195 = local read "Delay (ms)"() -> (w1776:i32)
        n1196 = call "serial write macro.vi"("String"=w1767, "Delay (ms)"=w1776, "VISA resource name"=w1773) -> ("read buffer"=w1774:string, "error out"=w1775:errorcluster, "VISA resource name out"=w1768:refnum<visa-resource-name>)
        n1197 = local write "read blue buffer"(w1774) -> ()
        n1198 = local write "Blue Error Out"(w1775) -> ()
        n1199 = local read "Delay (ms)"() -> (w1771:i32)
        n1200 = call "serial write macro.vi"("String"=w1766, "Delay (ms)"=w1771, "VISA resource name"=w1768) -> ("read buffer"=w1769:string, "error out"=w1770:errorcluster)  [unwired: 1 out]
        n1201 = local write "Blue Error Out"(w1770) -> ()
        n1202 = local write "read blue buffer"(w1769) -> ()
      }
      event "Blue Laser\nModulation\nPower (mW)": Value Change {
        n1203 = event-data() -> ()  [unwired: 1 in, 5 out]
        n1204 = local read "Blue Laser\nModulation\nPower (mW)"() -> (w1792:string)
        n1205 = local read "Blue Laser Modluation Mode"() -> (w1793:string)
        n1206 = case shown="\"Constant Power\"" w1793 {
          tunnel: w1792 -> [w1799 w1806]
          tunnel: [w1798 w1805] -> w1791
          frame "Constant Power" {
            # "Different command to change constant power instead of modulation power"
            n1207 = Decimal String To Number(string=w1799) -> (offset past number=w1804:i32)  [unwired: 2 in, 1 out]
            n1208 = Divide(x=w1804, y=1000) -> (x/y=w1802:dbl)
            n1209 = Number To Fractional String(number=w1802) -> (F-format string=w1800:string)  [unwired: 3 in]
            n1210 = Concatenate Strings("p ", w1800) -> (w1798:string)
          }
          frame Default {
            n1211 = Concatenate Strings("slmp ", w1806) -> (w1805:string)
          }
        }
        n1212 = local read "Delay (ms)"() -> (w1796:i32)
        n1213 = call "serial write macro.vi"("String"=w1791, "Delay (ms)"=w1796, "VISA resource name"=w1797) -> ("read buffer"=w1795:string, "error out"=w1794:errorcluster)  [unwired: 1 out]
        n1214 = local write "Blue Error Out"(w1794) -> ()
        n1215 = local write "read blue buffer"(w1795) -> ()
      }
      event "Send string\nto Blue Laser": Value Change {
        n1216 = event-data() -> ()  [unwired: 1 in, 5 out]
        n1217 = flat-sequence {
          tunnel: w1808 -> [w1813]
          frame #0 {
            n1218 = local read "Delay (ms)"() -> (w1810:i32)
            n1219 = call "serial write macro.vi"("String"="command string", "Delay (ms)"=w1810, "VISA resource name"=w1813) -> ("read buffer"=w1811:string, "error out"=→"Blue Error Out":errorcluster)  [unwired: 1 out]
            "read blue buffer" <- w1811
            n1220 = String Length(string=w1811) -> (length=→"length":i32)
            "command string sent" <- "command string"
          }
          frame #1 {
            n1221 = local write "Send string\nto Blue Laser"(FALSE ("Send string")) -> ()
          }
        }
      }
      event "Read Harvard": Value Change {
        n1222 = event-data() -> ()  [unwired: 1 in, 5 out]
        n1223 = Concatenate Strings("write buffer", "\r") -> (w1820:string)
        n1224 = VISA Write(VISA resource name=w1818, write buffer=w1820, error in (no error)=w1817) -> (VISA resource name out=w1829:refnum<visa-resource-name>, error out=w1828:errorcluster)  [unwired: 1 out]
        n1225 = stacked-sequence {
          tunnel: [w1832] -> w1827
          tunnel: w1829 -> [w1832]
          tunnel: w1828 -> [w1831]
          tunnel: [w1831] -> w1822
          frame #0 {
            n1226 = Wait (ms)(milliseconds to wait=50) -> ()  [unwired: 1 out]
          }
        }
        n1227 = property class="Instr"(reference=w1827, error in=w1822) -> (reference out=w1826:refnum<visa-resource-name>, error out=w1824:errorcluster, "Serial Settings:Number of Bytes at Serial Port"=w1825:u32)
        "Serial Settings:Number of Bytes at Serial Port" <- w1825
        n1228 = VISA Read(VISA resource name=w1826, byte count=w1825, error in (no error)=w1824) -> (read buffer=w1823:string)  [unwired: 3 out]
        "read buffer" <- w1823
        n1229 = Fract/Exp String To Number(string=w1823) -> ()  [unwired: 5 out]
      }
      event "+z", "-z": Value Change {
        n1230 = event-data() -> ()  [unwired: 1 in, 5 out]
        n1231 = flat-sequence {
          tunnel: w1833 -> [w1855]
          tunnel: w1834 -> [w1835]
          frame #0 {
            n1232 = call "Read Stage Position.vi"("error in"=w1855, "VISA resource name in"=w1835) -> ("Current Position"=w1840:cluster{dbl, dbl, dbl}, "error out"=w1853:errorcluster, "VISA resource name out"=w1854:refnum<visa-resource-name>)  [unwired: 1 out]
            n1233 = local read "Saved Stage Positions"() -> (w1864:dbl[][])
            n1234 = Divide(x="z nudge increment (um)", y=1000.0) -> (x/y=w1852:dbl)
            n1235 = Boolean To (0,1)(Boolean="+z") -> (0, 1=w1844:i16)
            n1236 = Boolean To (0,1)(Boolean="-z") -> (0, 1=w1845:i16)
            n1237 = Array Subset(array=w1864, index (row)=1 ("index"), length (row)=1 ("length"), index (col)=1 ("index"), length (col)=3 ("length")) -> (w1861:dbl[][])
            n1238 = Multiply(x=w1844, y=w1852) -> (x*y=w1848:dbl)
            n1239 = Multiply(x=w1845, y=w1852) -> (x*y=w1846:dbl)
            n1240 = Unbundle(w1840) -> (w1838:dbl, w1837:dbl, w1841:dbl)
            n1241 = Negate(x=w1846) -> (-x=w1847:dbl)
            n1242 = Reshape Array(w1861, 3 ("dimension size")) -> (w1859:dbl[])
            n1243 = Add(x=w1848, y=w1847) -> (x+y=w1849:dbl)
            n1244 = Array To Cluster(array=w1859) -> ()  [unwired: 1 out]
            n1245 = Add(x=w1849, y=w1841) -> (x+y=w1839:dbl)
            n1246 = Bundle(cluster=w1840, w1838, w1837, w1839) -> (w1836:cluster{dbl, dbl, dbl})
            n1247 = call "Set Stage Position.vi"("Position"=w1836, "error in"=w1853, "VISA resource name in"=w1854) -> ("error out"=w1858:errorcluster)  [unwired: 2 out]
            n1248 = local write "Stage Moving"(TRUE ("Stage Moving")) -> ()
            n1249 = local write "Stage Control Serial Error"(w1858) -> ()
          }
          frame #1 {
            n1250 = local write "Stage Moving"(FALSE ("Stage Moving")) -> ()
            n1251 = call <vilib>:"Beep.vi"() -> ()  [unwired: 3 in, 9 out]
          }
        }
      }
      event "Cal/Data Acq. Spot": Value Change {
        n1252 = event-data() -> ()  [unwired: 1 in, 5 out]
        n1253 = flat-sequence {
          tunnel: w1873 -> [w1877]
          tunnel: w1874 -> [w1878]
          tunnel: [w1878] -> w1870
          tunnel: [w1877] -> w1869
          tunnel: w1870 -> [w1883]
          tunnel: w1869 -> [w1882]
          tunnel: ["Cal @ (MHz)"] -> w1867
          tunnel: [w1887] -> w1871
          tunnel: w1867 -> [w1887]
          tunnel: w1871 -> [w1896]
          tunnel: ["W/ Offset 1"] -> w1868
          tunnel: w1871 -> [w1917]
          tunnel: w1868 -> [w1915]
          frame #0 {
            n1254 = property on="Sample Channel\nFlow" class="Bool (strict)"("Val(Sgnl)"="Daq spot flow on") -> ()  [unwired: 2 in, 2 out]
            n1255 = Wait (ms)(milliseconds to wait=u32 250) -> ()  [unwired: 1 out]
          }
          frame #1 {
            n1256 = local read "Saved Stage Positions"() -> (w1880:dbl[][])
            n1257 = property on="Trap Delta (MHz)" class="DigNum (strict)"("Val(Sgnl)"="Cal @ (MHz)") -> ()  [unwired: 2 in, 2 out]
            n1258 = local write "Stage Moving"(TRUE ("Stage Moving")) -> ()
            n1259 = call "move to saved stage position.vi"("error in"=w1882, "Stage VISA resource name in"=w1883, "Position"="Cal Stage Position", "Saved Stage Positions"=w1880) -> ("error out"=w1881:errorcluster)  [unwired: 1 out]
            n1260 = local write "Stage Control Serial Error"(w1881) -> ()
          }
          frame #2 {
            n1261 = local write "Stage Moving"(FALSE ("Stage Moving")) -> ()
            n1262 = property on="Sample Channel\nFlow" class="Bool (strict)"("Val(Sgnl)"="Flow ON during cal?") -> ()  [unwired: 2 in, 2 out]
            n1263 = call <vilib>:"Beep.vi"() -> ()  [unwired: 3 in, 9 out]
          }
          frame #3 {
            n1264 = Wait (ms)(milliseconds to wait=u32 1000) -> ()  [unwired: 1 out]
          }
          frame #4 {
            n1265 = property on="Save Calibration" class="Bool (strict)"("Val(Sgnl)"=TRUE ("Value (Signaling)")) -> ()  [unwired: 2 in, 2 out]
          }
          frame #5 {
            n1266 = Wait (ms)(milliseconds to wait=u32 2000) -> ()  [unwired: 1 out]
          }
          frame #6 {
            # "Check to see if \nsaving done"
            n1267 = while {
              stop <- w1892 stop-if-true
              n1268 = local read "Saving..."() -> (w1893:bool)
              n1269 = Wait (ms)(milliseconds to wait=u32 100) -> ()  [unwired: 1 out]
              n1270 = Not(x=w1893) -> (.not. x?=w1892:bool)
            }
          }
          frame #7 {
            n1271 = case shown="True" "W/ Offset 1" {
              tunnel: w1896 -> [_ w1897]
              frame False {
              }
              frame True {
                n1272 = stacked-sequence {
                  tunnel: w1897 -> [_ _ _ _ _ _ _ w1914]
                  frame #0 {
                    n1273 = property on="Trap Delta (MHz)" class="DigNum (strict)"("Val(Sgnl)"="Offset 1 Start (MHz)") -> ()  [unwired: 2 in, 2 out]
                    n1274 = Replace Array Subset(array=u32[] [0] ("Index Values"), new element="Offset 1 Set", index=0) -> (w1898:u32[])
                    n1275 = property on="Saved AOD Raster Scan Parameter Sets" class="Arr (strict)"("Index Values"=w1898) -> ()  [unwired: 2 in, 2 out]
                  }
                  frame #1 {
                    n1276 = Wait (ms)(milliseconds to wait=u32 200) -> ()  [unwired: 1 out]
                  }
                  frame #2 {
                    n1277 = property on="Load parameters" class="Bool (strict)"("Val(Sgnl)"=TRUE ("Value (Signaling)")) -> ()  [unwired: 2 in, 2 out]
                  }
                  frame #3 {
                    n1278 = Wait (ms)(milliseconds to wait=u32 200) -> ()  [unwired: 1 out]
                  }
                  frame #4 {
                    n1279 = property on="Trap Raster Scan" class="Bool (strict)"("Val(Sgnl)"=TRUE ("Value (Signaling)")) -> ()  [unwired: 2 in, 2 out]
                  }
                  frame #5 {
                    n1280 = Wait (ms)(milliseconds to wait=u32 2000) -> ()  [unwired: 1 out]
                  }
                  frame #6 {
                    n1281 = while {
                      stop <- w1911 stop-if-true
                      n1282 = local read "Raster Scanning..."() -> (w1913:bool)
                      n1283 = local read "Saving..."() -> (w1909:bool)
                      n1284 = Wait (ms)(milliseconds to wait=u32 100) -> ()  [unwired: 1 out]
                      n1285 = Not(x=w1909) -> (.not. x?=w1908:bool)
                      n1286 = Not(x=w1913) -> (.not. x?=w1910:bool)
                      n1287 = And(x=w1910, y=w1908) -> (x .and. y?=w1911:bool)
                    }
                  }
                  frame #7 {
                    n1288 = property on="Trap Delta (MHz)" class="DigNum (strict)"("Val(Sgnl)"=w1914) -> ()  [unwired: 2 in, 2 out]
                  }
                }
              }
            }
          }
          frame #8 {
            n1289 = local read "Save ave N"() -> (w1916:dbl)
            n1290 = case shown="False" "W/ Offset 2" {
              tunnel: w1917 -> [_ w1924]
              tunnel: w1916 -> [_ w1923]
              tunnel: w1915 -> [w1919 _]
              frame False {
                n1291 = case shown="False" w1919 {
                  frame False {
                    n1292 = Multiply(x="Cal read wait (s)", y=u32 1000 ("milliseconds to wait")) -> (x*y=w1921:u32)
                    n1293 = Wait (ms)(milliseconds to wait=w1921) -> ()  [unwired: 1 out]
                  }
                  frame True {
                  }
                }
              }
              frame True {
                n1294 = stacked-sequence {
                  tunnel: w1924 -> [_ _ _ _ _ _ _ _ _ w1945 _ _]
                  tunnel: w1923 -> [_ _ _ _ _ _ _ _ _ w1943 _ _]
                  frame #0 {
                    n1295 = property on="Save ave N" class="DigNum (strict)"("Val(Sgnl)"=1.0 ("Value (Signaling)")) -> ()  [unwired: 2 in, 2 out]
                  }
                  frame #1 {
                    n1296 = Wait (ms)(milliseconds to wait=u32 500) -> ()  [unwired: 1 out]
                  }
                  frame #2 {
                    n1297 = property on="Trap Delta (MHz)" class="DigNum (strict)"("Val(Sgnl)"="Offset 2 Start (MHz)") -> ()  [unwired: 2 in, 2 out]
                    n1298 = Replace Array Subset(array=u32[] [0] ("Index Values"), new element="Offset 2 Set", index=0) -> (w1929:u32[])
                    n1299 = property on="Saved AOD Raster Scan Parameter Sets" class="Arr (strict)"("Index Values"=w1929) -> ()  [unwired: 2 in, 2 out]
                  }
                  frame #3 {
                    n1300 = Wait (ms)(milliseconds to wait=u32 500) -> ()  [unwired: 1 out]
                  }
                  frame #4 {
                    n1301 = property on="Load parameters" class="Bool (strict)"("Val(Sgnl)"=TRUE ("Value (Signaling)")) -> ()  [unwired: 2 in, 2 out]
                  }
                  frame #5 {
                    n1302 = Wait (ms)(milliseconds to wait=u32 500) -> ()  [unwired: 1 out]
                  }
                  frame #6 {
                    n1303 = property on="Trap Raster Scan" class="Bool (strict)"("Val(Sgnl)"=TRUE ("Value (Signaling)")) -> ()  [unwired: 2 in, 2 out]
                  }
                  frame #7 {
                    n1304 = Wait (ms)(milliseconds to wait=u32 2000) -> ()  [unwired: 1 out]
                  }
                  frame #8 {
                    n1305 = while {
                      stop <- w1938 stop-if-true
                      n1306 = local read "Raster Scanning..."() -> (w1941:bool)
                      n1307 = local read "Saving..."() -> (w1939:bool)
                      n1308 = Wait (ms)(milliseconds to wait=u32 100) -> ()  [unwired: 1 out]
                      n1309 = Not(x=w1939) -> (.not. x?=w1937:bool)
                      n1310 = Not(x=w1941) -> (.not. x?=w1940:bool)
                      n1311 = And(x=w1940, y=w1937) -> (x .and. y?=w1938:bool)
                    }
                  }
                  frame #9 {
                    n1312 = property on="Trap Delta (MHz)" class="DigNum (strict)"("Val(Sgnl)"=w1945) -> ()  [unwired: 2 in, 2 out]
                    n1313 = property on="Saved AOD Raster Scan Parameter Sets" class="Arr (strict)"("Index Values"=u32[] [0]) -> ()  [unwired: 2 in, 2 out]
                    n1314 = property on="Save ave N" class="DigNum (strict)"("Val(Sgnl)"=w1943) -> ()  [unwired: 2 in, 2 out]
                  }
                  frame #10 {
                    n1315 = Wait (ms)(milliseconds to wait=u32 500) -> ()  [unwired: 1 out]
                  }